vi "UHR-Fleezers Control (host) - 10.7.vi"() -> ()   [LabVIEW 2010] (continued)
            n1703 = case shown="False" w7659 {
              tunnel: w7658 -> [w7665 w7679]
              tunnel: "Chemyx Syringe Pump Serial Port" -> [w7662 w7678]
              frame False {
                n1704 = flat-sequence {
                  tunnel: w7662 -> [w7666]
                  tunnel: [w7666] -> w7663
                  tunnel: w7665 -> [_]
                  tunnel: [w7669] -> w7664
                  tunnel: w7663 -> [w7669]
                  tunnel: w7664 -> [w7670]
                  tunnel: [w7670] -> w7660
                  tunnel: [w7672] -> w7661
                  tunnel: w7660 -> [w7672]
                  tunnel: w7661 -> [w7674]
                  frame #0 {
                    n1705 = call "Write to pump.vi"("string"="enter pump3", "VISA resource name"=w7666) -> ()  [unwired: 1 out]
                  }
                  frame #1 {
                    n1706 = local read "Pump pause delay (ms)"() -> (w7668:u32)
                    n1707 = Wait (ms)(milliseconds to wait=w7668) -> ()  [unwired: 1 out]
                  }
                  frame #2 {
                    n1708 = call "Write to pump.vi"("string"="stop", "VISA resource name"=w7670) -> ()  [unwired: 1 out]
                  }
                  frame #3 {
                    n1709 = Wait (ms)(milliseconds to wait=u32 0) -> ()  [unwired: 1 out]
                  }
                  frame #4 {
                    n1710 = call "Write to pump.vi"("string"="stop", "VISA resource name"=w7674) -> ()  [unwired: 1 out]
                  }
                }
              }
              frame True {
                n1711 = flat-sequence {
                  tunnel: w7678 -> [w7688]
                  tunnel: w7679 -> [w7683]
                  tunnel: w7679 -> [w7690]
                  tunnel: w7678 -> [w7691]
                  tunnel: [w7691] -> w7676
                  tunnel: [w7694] -> w7677
                  tunnel: w7676 -> [w7694]
                  tunnel: w7677 -> [w7695]
                  frame #0 {
                    n1712 = local read "All Pump Parameters"() -> (w7682:T5)
                    n1713 = Unbundle By Name(w7682) -> ("Pump 3"=w7689:T51)
                    n1714 = call "Set pump parameters.vi"("Pump write delay (ms)"=w7683, "Volume (uL)"="Ch 3 Inject Volume (uL)", "Rate (uL/h)"="Ch 3 Inject Rate (ul/h)", "Units"=4.0, "Pump #"=3.0, "Pump Parameters In"=w7689, "VISA resource name"=w7688) -> ("Pump Parameters Out"=w7681:T51)  [unwired: 3 in]
                    n1715 = Bundle By Name(cluster=w7682, "Pump 3"=w7681) -> (w7680:T5)
                    n1716 = local write "All Pump Parameters"(w7680) -> ()
                  }
                  frame #1 {
                    n1717 = Wait (ms)(milliseconds to wait=w7690) -> ()  [unwired: 1 out]
                  }
                  frame #2 {
                    n1718 = call "Write to pump.vi"("string"="start", "VISA resource name"=w7691) -> ()  [unwired: 1 out]
                  }
                  frame #3 {
                    n1719 = Wait (ms)(milliseconds to wait=u32 500) -> ()  [unwired: 1 out]
                  }
                  frame #4 {
                    n1720 = call "Write to pump.vi"("string"="start", "VISA resource name"=w7695) -> ()  [unwired: 1 out]
                  }
                }
              }
            }
          }
          frame Enabled {
            n1721 = call "hamilton_controller.vi"("Open?"=w7697, "valve"=enum16{"A", "B", "C", "D", "ALL"}."A", "action"=T23."MOVE VALVE") -> ()  [unwired: 8 in, 1 out]
          }
        }
      }
      event "Inject Valve B": Value Change {
        n1722 = event-data() -> ()  [unwired: 7 out]
        n1723 = disable-structure shown="Enabled" {
          disable-tunnel: "Inject Valve B" -> [w7701 w7721]
          frame Disabled {
            n1724 = local read "Pump write delay (ms)"() -> (w7703:dbl)
            n1725 = flat-sequence {
              tunnel: w7702 -> [w7716]
              tunnel: w7703 -> [w7712]
              tunnel: w7701 -> [_]
              tunnel: w7703 -> [w7718]
              tunnel: w7702 -> [w7719]
              frame #0 {
                n1726 = local read "All Pump Parameters"() -> (w7711:T5)
                n1727 = Multiply(x=60.0, y="Flush Center Ch Rate (ul/m)") -> (x*y=w7708:dbl)
                n1728 = Unbundle By Name(w7711) -> ("Pump 2"=w7717:T51)
                n1729 = call "Set pump parameters.vi"("Pump write delay (ms)"=w7712, "Volume (uL)"="Flush Center Ch Volume (uL)", "Rate (uL/h)"=w7708, "Units"=3.0, "Pump #"=2.0, "Pump Parameters In"=w7717, "VISA resource name"=w7716) -> ("Pump Parameters Out"=w7710:T51)  [unwired: 3 in]
                n1730 = Bundle By Name(cluster=w7711, "Pump 2"=w7710) -> (w7709:T5)
                n1731 = local write "All Pump Parameters"(w7709) -> ()
                n1732 = Add(x="Flush Center Ch Volume (uL)", y="Total Volume\nFlushed (uL)") -> (x+y=w7705:dbl)
                n1733 = local write "Total Volume\nFlushed (uL)"(w7705) -> ()
              }
              frame #1 {
                n1734 = Wait (ms)(milliseconds to wait=w7718) -> ()  [unwired: 1 out]
              }
              frame #2 {
                n1735 = call "Write to pump.vi"("string"="start", "VISA resource name"=w7719) -> ()  [unwired: 1 out]
              }
            }
            n1736 = local read "Chemyx Syringe Pump Serial Port"() -> (w7702:refnum<visa-resource-name>)
          }
          frame Enabled {
            n1737 = call "hamilton_controller.vi"("Open?"=w7721, "valve"=enum16{"A", "B", "C", "D", "ALL"}."B", "action"=T23."MOVE VALVE") -> ()  [unwired: 8 in, 1 out]
          }
        }
      }
      event "Sample Channel Flow": Value Change {
        n1738 = event-data() -> ()  [unwired: 7 out]
        n1739 = call "hamilton_controller.vi"("Open?"="Sample Channel Flow", "valve"=enum16{"A", "B", "C", "D", "ALL"}."C", "action"=T23."MOVE VALVE") -> ()  [unwired: 8 in, 1 out]
      }
      event "Flip Green Filter": Value Change {
        n1740 = event-data() -> ()  [unwired: 7 out]
        n1741 = Not(x="Flip Green Filter") -> (.not. x?=w7727:bool)
        n1742 = local write "Flip Green Filter"(w7727) -> ()
        n1743 = flat-sequence {
          tunnel: w7735 -> [w7740]
          tunnel: w7734 -> [w7739]
          tunnel: [w7737] -> w7732
          tunnel: [w7736] -> w7731
          tunnel: [w7780] -> w7730
          tunnel: w7732 -> [w7780]
          tunnel: [w7779] -> w7729
          tunnel: w7731 -> [w7779]
          tunnel: w7730 -> [w7784]
          tunnel: w7729 -> [w7783]
          tunnel: [w7782] -> w7733
          frame #0 {
            n1744 = xnode "Read/Write Control"("FPGA VI Reference In"=w7740, "error in"=w7739, "Green Filter Flipper"=TRUE) -> ("FPGA VI Reference Out"=w7737:T19, "error out"=w7736:errorcluster)
          }
          frame #1 {
            n1745 = Wait (ms)(milliseconds to wait=u32 100) -> ()  [unwired: 1 out]
          }
          frame #2 {
            n1746 = xnode "Read/Write Control"("FPGA VI Reference In"=w7784, "error in"=w7783, "Green Filter Flipper"=FALSE) -> ("error out"=w7782:errorcluster)  [unwired: 1 out]
          }
        }
      }
      event "Pump 1 contents", "Pump 3 contents": Value Change {
        n1747 = event-data() -> ()  [unwired: 7 out]
        n1748 = local read "Pump 1 contents"() -> (→"Pump 1 cont disp":string)
        n1749 = local read "Pump 3 contents"() -> (→"Pump 3 cont disp":string)
      }
      event "Reset Trap Pos. FB": Value Change {
        n1750 = event-data() -> ()  [unwired: 7 out]
        n1751 = xnode "Read/Write Control"("FPGA VI Reference In"=w7828, "error in"=w7827, "Trap Pos. FB Reset"="Reset Trap Pos. FB") -> ()  [unwired: 2 out]
      }
      event "Trap Pos. FB ON": Value Change {
        n1752 = event-data() -> ()  [unwired: 7 out]
        n1753 = xnode "Read/Write Control"("FPGA VI Reference In"=w7869, "error in"=w7868, "Force feedback"="Trap Pos. FB ON") -> ()  [unwired: 2 out]
      }
      event "Trap Pos. FB Range", "Trap Pos. FB Gains", "Trap Pos. FB Mult Factor", "Trap Pos. FB Offset Factor", "Trap Pos FB Negate Action", "Trap Pos FB Monitor\nT1 or T2": Value Change {
        n1754 = event-data() -> ()  [unwired: 7 out]
        n1755 = xnode "Read/Write Control"("FPGA VI Reference In"=w7916, "error in"=w7915, "Trap Pos. FB Range"="Trap Pos. FB Range", "Trap Pos. FB Gains"="Trap Pos. FB Gains", "Trap Pos. FB Mult Factor"="Trap Pos. FB Mult Factor", "Trap Pos. FB Offset Factor"="Trap Pos. FB Offset Factor", "Trap Pos FB Negate Action"="Trap Pos FB Negate Action", "Trap Pos FB Monitor T1 or T2"="Trap Pos FB Monitor\nT1 or T2", "AI1 X Scale"="Trap Pos. AI1 X Pre-scale") -> ()  [unwired: 2 out]
      }
      event "Trap Pos FB SP": Value Change {
        n1756 = event-data() -> ()  [unwired: 7 out]
        n1757 = xnode "Read/Write Control"("FPGA VI Reference In"=w8104, "error in"=w8103, "Trap Pos. FB SP"="Trap Pos FB SP") -> ()  [unwired: 2 out]
      }
      event "Set SP to Reading": Value Change {
        n1758 = event-data() -> ()  [unwired: 7 out]
        n1759 = local read "Trap Pos FB Monitor\nT1 or T2"() -> (w8157:bool)
        n1760 = local read "Trap X AI1 (DMA)"() -> (w8160:T13)
        n1761 = local read "Trap X (AI1)"() -> (w8163:T10)
        n1762 = Unbundle By Name(w8163) -> ("Trap 1"=w8162:fxp<+/-,16,1>, "Trap 2"=w8161:fxp<+/-,16,1>)
        n1763 = Unbundle By Name(w8160) -> ("Set 1"=w8159:fxp<+/-,16,1>, "Set 2"=w8158:fxp<+/-,16,1>)
        n1764 = Select(t=w8162, s=w8157, f=w8161) -> (s? t:f=w8156:fxp<+/-,16,1>)
        n1765 = Select(t=w8159, s=w8157, f=w8158) -> (s? t:f=w8155:fxp<+/-,16,1>)
        n1766 = Not(x="Set SP Using...") -> (.not. x?=w8150:bool)
        n1767 = Select(t=w8156, s=w8150, f=w8155) -> (s? t:f=w8151:fxp<+/-,16,1>)
        n1768 = xnode "Read/Write Control"("FPGA VI Reference In"=w8153, "error in"=w8152, "Trap Pos. FB SP"=w8151) -> ()  [unwired: 2 out]
        n1769 = local write "Trap Pos FB SP"(w8151) -> ()
      }
      event "Trap Pos. FB Out Scale 2^n": Value Change {
        n1770 = event-data() -> ()  [unwired: 7 out]
        n1771 = Scale By Power Of 2(n="Trap Pos. FB Out Scale 2^n", x=ext 1.0) -> (x*2^n=w8210:ext)
        n1772 = property on="Trap Pos. FB Mult Factor" class="DigNum (strict)"("Val(Sgnl)"=w8210) -> ()  [unwired: 2 in, 2 out]
      }
      event "Trap Pos FB Int Count": Value Change {
        n1773 = event-data() -> ()  [unwired: 7 out]
        n1774 = xnode "Read/Write Control"("FPGA VI Reference In"=w8215, "error in"=w8214, "Trap Pos FB Int Count"="Trap Pos FB Int Count") -> ()  [unwired: 2 out]
      }
    }
    "error out 2" <- w4481
    n1775 = node-c288() -> ()  [unwired: 1 in, 1 out]
  }
  n1776 = timed-loop "Run Scripts, including: stage motion" {
    timing: w68 -> [_]
    timing-out: [_] -> w67
    tunnel: w16 -> [_]
    stop <- w8254 stop-if-true
    n1777 = node-c288() -> ()  [unwired: 1 in, 1 out]
    n1778 = event shown="[11] \"Got ADig bead\": Value Change" {
      selector: _ -> [_ _ _ _ _ _ _ _ _ _ _ _ _ _ _ _ _]
      dyn-events: _ -> [_ _ _ _ _ _ _ _ _ _ _ _ _ _ _ _ _]
      timeout: 50 -> [_ _ _ _ _ _ _ _ _ _ _ _ _ _ _ _ _]
      tunnel: ["Set Position" "Move to Position" "Move Cap. 1 (DNA Top)" _ "Move Cap. 2 (ADig Bot)" _ "Cal/Data Acq. Spot" "Dump Beads" "Dip for Protein" _ _ "Got ADig bead" "Got DNA bead" "Take Stepping Data" _ "Take Detection Laser\nImage" _] -> _
      tunnel: [_ _ _ _ _ _ _ _ _ _ _ _ _ _ _ _ w8636] -> w8254
      event "Set Position", "Set Position 2", "Set Position 3", "Set Position 4", "Set Position 5", "Set Position 1": Value Change {
        n1779 = event-data() -> ()  [unwired: 1 in, 5 out]
        n1780 = Build Array("Set Position 1", "Set Position 2", "Set Position 3", "Set Position 4", "Set Position 5") -> (w8273:bool[])
        n1781 = Boolean Array To Number(Boolean array=w8273) -> (number=w8272:u32)
        n1782 = Logarithm Base 2(1:w8272) -> (0:w8264:dbl)
        n1783 = call "CONEX_FUNCTIONAL_GLOBAL.vi"("Command"=T22."GET POS") -> ("Current Position"=w8257:dbl[])  [unwired: 8 in, 2 out]
        n1784 = Decrement(x="Position") -> (x-1=w8262:dbl)
        n1785 = Greater Or Equal?(x=w8264, y=0.0) -> (x >= y?=w8265:bool)
        n1786 = Select(t=w8264, s=w8265, f=w8262) -> (s? t:f=w8261:dbl)
        n1787 = Increment(x=w8261) -> (x+1=w8260:dbl)
        n1788 = Build Array (concatenate)(w8260, w8257) -> (w8259:dbl[])
        n1789 = Replace Array Subset(array="Saved Stage Positions", new element=w8259, index (row)=w8261) -> (w8274:dbl[][])  [unwired: 1 in]
        n1790 = local write "Saved Stage Positions"(w8274) -> ()
      }
      event "Move to Position": Value Change {
        n1791 = event-data() -> ()  [unwired: 1 in, 5 out]
        n1792 = flat-sequence {
          frame #0 {
            n1793 = local read "Position"() -> (w8289:dbl)
            n1794 = local read "Saved Stage Positions"() -> (w8287:dbl[][])
            n1795 = Decrement(x=w8289) -> (x-1=w8286:dbl)
            n1796 = Array Subset(array=w8287, index (row)=w8286, length (row)=1 ("length"), index (col)=1 ("index"), length (col)=3 ("length")) -> (w8283:dbl[][])
            n1797 = Reshape Array(w8283, 3 ("dimension size")) -> (w8279:dbl[])
            n1798 = local write "Stage Moving"(TRUE ("Stage Moving")) -> ()
            n1799 = call "CONEX_FUNCTIONAL_GLOBAL.vi"("Axis"=enum16{"X", "Y", "Z", "XY", "XZ", "YZ", "XYZ"}."XYZ", "Position"=w8279, "Command"=T22."ABS MOVE") -> ()  [unwired: 6 in, 3 out]
          }
          frame #1 {
            n1800 = call <vilib>:"Beep.vi"() -> ()  [unwired: 3 in, 9 out]
            n1801 = local write "Stage Moving"(FALSE ("Stage Moving")) -> ()
          }
        }
      }
      event "Move Cap. 1 (DNA Top)": Value Change {
        n1802 = event-data() -> ()  [unwired: 1 in, 5 out]
        n1803 = local write "Move Cap. 1 (DNA Top)"(FALSE ("Move Cap. 1 (DNA Right)")) -> ()
        n1804 = flat-sequence {
          tunnel: ["Cap 1 Samp Flow ON"] -> w8292
          tunnel: w8292 -> [w8311]
          tunnel: [w8311] -> w8291
          tunnel: w8291 -> [w8312]
          frame #0 {
            n1805 = local read "Saved Stage Positions"() -> (w8305:dbl[][])
            n1806 = Array Subset(array=w8305, index (row)=0 ("index"), length (row)=1 ("length"), index (col)=1 ("index"), length (col)=3 ("length")) -> (w8302:dbl[][])
            n1807 = Reshape Array(w8302, 3 ("dimension size")) -> (w8296:dbl[])
            n1808 = case "start flow in central channel to wash" shown="True" "Cap 1 Samp Flow ON" {
              frame False {
              }
              frame True {
                n1809 = call "hamilton_controller.vi"("Open?"=TRUE, "valve"=enum16{"A", "B", "C", "D", "ALL"}."C", "action"=T23."MOVE VALVE") -> ()  [unwired: 8 in, 1 out]
              }
            }
            n1810 = call "CONEX_FUNCTIONAL_GLOBAL.vi"("Axis"=enum16{"X", "Y", "Z", "XY", "XZ", "YZ", "XYZ"}."XYZ", "Position"=w8296, "Command"=T22."ABS MOVE") -> ()  [unwired: 6 in, 3 out]
            n1811 = local write "Stage Moving"(TRUE ("Stage Moving")) -> ()
          }
          frame #1 {
            # "should replace this frame\nwith code that \ncontinuously polls the\nCONEX controllers to\ndetermine when the \nmotors have finished \nmoving. once the move \nis finished, proceed to\nnext frame"
            n1812 = Wait (ms)(milliseconds to wait=u32 5000) -> ()  [unwired: 1 out]
          }
          frame #2 {
            n1813 = local write "Stage Moving"(FALSE ("Stage Moving")) -> ()
            n1814 = case "stop flow" shown="False" w8312 {
              frame False {
              }
              frame True {
                n1815 = call "hamilton_controller.vi"("Open?"=FALSE, "valve"=enum16{"A", "B", "C", "D", "ALL"}."C", "action"=T23."MOVE VALVE") -> ()  [unwired: 8 in, 1 out]
              }
            }
            n1816 = case shown="True" TRUE {
              tunnel: "Cap 1 T ON" -> [w8321 w8322]
              frame False {
                n1817 = property on="Trap 1 (ON/OFF)" class="Bool (strict)"("Val(Sgnl)"=w8321) -> ()  [unwired: 2 in, 2 out]
              }
              frame True {
                n1818 = property on="Trap 2 (ON/OFF)" class="Bool (strict)"("Val(Sgnl)"=w8322) -> ()  [unwired: 2 in, 2 out]
              }
            }
            n1819 = call <vilib>:"Beep.vi"() -> ()  [unwired: 3 in, 9 out]
            n1820 = case shown="True" "Cap 1 Flow ON" {
              frame False {
              }
              frame True {
                n1821 = property on="Inject Top" class="Bool (strict)"("Val(Sgnl)"=TRUE ("Value (Signaling)")) -> ()  [unwired: 2 in, 2 out]
              }
            }
          }
        }
      }
      event Timeout {
        n1822 = event-data() -> ()  [unwired: 1 in, 2 out]
      }
      event "Move Cap. 2 (ADig Bot)": Value Change {
        n1823 = event-data() -> ()  [unwired: 1 in, 5 out]
        n1824 = local write "Move Cap. 2 (ADig Bot)"(FALSE ("Move Cap. 2 (ADig Left)")) -> ()
        n1825 = flat-sequence {
          tunnel: ["Cap 2 Samp Flow ON"] -> w8324
          tunnel: w8324 -> [w8343]
          tunnel: [w8343] -> w8323
          tunnel: w8323 -> [w8344]
          frame #0 {
            n1826 = local read "Saved Stage Positions"() -> (w8337:dbl[][])
            n1827 = case shown="True" "Cap 2 Samp Flow ON" {
              frame False {
              }
              frame True {
                n1828 = call "hamilton_controller.vi"("Open?"=TRUE, "valve"=enum16{"A", "B", "C", "D", "ALL"}."C", "action"=T23."MOVE VALVE") -> ()  [unwired: 8 in, 1 out]
              }
            }
            n1829 = Array Subset(array=w8337, index (row)=1 ("index"), length (row)=1 ("length"), index (col)=1 ("index"), length (col)=3 ("length")) -> (w8334:dbl[][])
            n1830 = Reshape Array(w8334, 3 ("dimension size")) -> (w8328:dbl[])
            n1831 = local write "Stage Moving"(TRUE ("Stage Moving")) -> ()
            n1832 = call "CONEX_FUNCTIONAL_GLOBAL.vi"("Axis"=enum16{"X", "Y", "Z", "XY", "XZ", "YZ", "XYZ"}."XYZ", "Position"=w8328, "Command"=T22."ABS MOVE") -> ()  [unwired: 6 in, 3 out]
          }
          frame #1 {
            n1833 = Wait (ms)(milliseconds to wait=u32 5000) -> ()  [unwired: 1 out]
          }
          frame #2 {
            n1834 = local write "Stage Moving"(FALSE ("Stage Moving")) -> ()
            n1835 = case shown="True" TRUE {
              tunnel: "Cap 2 T ON" -> [w8353 w8354]
              frame False {
                n1836 = property on="Trap 2 (ON/OFF)" class="Bool (strict)"("Val(Sgnl)"=w8353) -> ()  [unwired: 2 in, 2 out]
              }
              frame True {
                n1837 = property on="Trap 1 (ON/OFF)" class="Bool (strict)"("Val(Sgnl)"=w8354) -> ()  [unwired: 2 in, 2 out]
              }
            }
            n1838 = call <vilib>:"Beep.vi"() -> ()  [unwired: 3 in, 9 out]
            n1839 = case shown="True" w8344 {
              frame False {
              }
              frame True {
                n1840 = call "hamilton_controller.vi"("Open?"=FALSE, "valve"=enum16{"A", "B", "C", "D", "ALL"}."C", "action"=T23."MOVE VALVE") -> ()  [unwired: 8 in, 1 out]
              }
            }
            n1841 = case shown="True" "Cap 2 Flow ON" {
              frame False {
              }
              frame True {
                n1842 = property on="Inject Bottom" class="Bool (strict)"("Val(Sgnl)"=TRUE ("Value (Signaling)")) -> ()  [unwired: 2 in, 2 out]
              }
            }
          }
        }
      }
      event "+z", "-z": Value Change {
        n1843 = event-data() -> ()  [unwired: 1 in, 5 out]
        n1844 = flat-sequence {
          frame #0 {
            w8356 = 0.0 ("element")
            n1845 = Divide(x="z nudge increment (um)", y=1000.0) -> (x/y=w8369:dbl)
            n1846 = Boolean To (0,1)(Boolean="+z") -> (0, 1=w8362:i16)
            n1847 = Boolean To (0,1)(Boolean="-z") -> (0, 1=w8363:i16)
            n1848 = Multiply(x=w8362, y=w8369) -> (x*y=w8366:dbl)
            n1849 = Multiply(x=w8363, y=w8369) -> (x*y=w8364:dbl)
            n1850 = Negate(x=w8364) -> (-x=w8365:dbl)
            n1851 = Add(x=w8366, y=w8365) -> (x+y=w8357:dbl)
            n1852 = Build Array(w8356, w8356, w8357) -> (w8355:dbl[])
            n1853 = call "CONEX_FUNCTIONAL_GLOBAL.vi"("Axis"=enum16{"X", "Y", "Z", "XY", "XZ", "YZ", "XYZ"}."Z", "Position"=w8355, "Command"=T22."REL MOVE") -> ()  [unwired: 6 in, 3 out]
            n1854 = local write "Stage Moving"(TRUE ("Stage Moving")) -> ()
          }
          frame #1 {
            n1855 = local write "Stage Moving"(FALSE ("Stage Moving")) -> ()
            n1856 = call <vilib>:"Beep.vi"() -> ()  [unwired: 3 in, 9 out]
          }
        }
      }
      event "Cal/Data Acq. Spot": Value Change {
        # "wait for calibration file\nto be written"
        # "signal save cal true\nthis tells the data \nacquisition loop to\nstart sending the data\nto a calibration file"
        # "separate traps to\nthe desired trap delta"
        # "move stage to data acquisition spot"
        # "CHANGE FISH FOR TETHER BACK\nTO TRUE VALUE HERE."
        n1857 = event-data() -> ()  [unwired: 1 in, 5 out]
        n1858 = flat-sequence {
          tunnel: ["Cal @ (MHz)"] -> w8372
          tunnel: w8372 -> [w8394]
          tunnel: w8372 -> [w8415]
          frame #0 {
            n1859 = local read "Saved Stage Positions"() -> (w8380:dbl[][])
            n1860 = Array Subset(array=w8380, index (row)=2 ("index"), length (row)=1 ("length"), index (col)=1 ("index"), length (col)=3 ("length")) -> (w8383:dbl[][])
            n1861 = Reshape Array(w8383, 3 ("dimension size")) -> (w8376:dbl[])
            n1862 = local write "Stage Moving"(TRUE ("Stage Moving")) -> ()
            n1863 = call "CONEX_FUNCTIONAL_GLOBAL.vi"("Axis"=enum16{"X", "Y", "Z", "XY", "XZ", "YZ", "XYZ"}."XYZ", "Position"=w8376, "Command"=T22."ABS MOVE") -> ()  [unwired: 6 in, 3 out]
          }
          frame #1 {
            n1864 = property on="Trap Delta (MHz)" class="DigNum (strict)"("Val(Sgnl)"="Cal @ (MHz)") -> ()  [unwired: 2 in, 2 out]
            n1865 = local write "Stage Moving"(FALSE ("Stage Moving")) -> ()
            n1866 = call <vilib>:"Beep.vi"() -> ()  [unwired: 3 in, 9 out]
          }
          frame #2 {
            n1867 = Wait (ms)(milliseconds to wait=u32 100) -> ()  [unwired: 1 out]
          }
          frame #3 {
            n1868 = property on="Save Calibration" class="Bool (strict)"("Val(Sgnl)"=TRUE ("Value (Signaling)")) -> ()  [unwired: 2 in, 2 out]
          }
          frame #4 {
            n1869 = Wait (ms)(milliseconds to wait=u32 4000) -> ()  [unwired: 1 out]
          }
          frame #5 {
            n1870 = while {
              stop <- w8391 stop-if-true
              n1871 = local read "Saving..."() -> (w8392:bool)
              n1872 = Wait (ms)(milliseconds to wait=u32 100) -> ()  [unwired: 1 out]
              n1873 = Not(x=w8392) -> (.not. x?=w8391:bool)
            }
          }
          frame #6 {
            n1874 = case shown="True" "W/ Offset 1" {
              tunnel: w8394 -> [_ w8396]
              frame False {
              }
              frame True {
                n1875 = stacked-sequence {
                  tunnel: w8396 -> [_ _ _ _ _ _ _ w8413]
                  frame #0 {
                    n1876 = property on="Trap Delta (MHz)" class="DigNum (strict)"("Val(Sgnl)"="Offset 1 Start (MHz)") -> ()  [unwired: 2 in, 2 out]
                    n1877 = Replace Array Subset(array=u32[] [0] ("Index Values"), new element="Offset 1 Set", index=0) -> (w8397:u32[])
                    n1878 = property on="Saved AOD Raster Scan Parameter Sets" class="Arr (strict)"("Index Values"=w8397) -> ()  [unwired: 2 in, 2 out]
                  }
                  frame #1 {
                    n1879 = Wait (ms)(milliseconds to wait=u32 200) -> ()  [unwired: 1 out]
                  }
                  frame #2 {
                    n1880 = property on="Load parameters" class="Bool (strict)"("Val(Sgnl)"=TRUE ("Value (Signaling)")) -> ()  [unwired: 2 in, 2 out]
                  }
                  frame #3 {
                    n1881 = Wait (ms)(milliseconds to wait=u32 200) -> ()  [unwired: 1 out]
                  }
                  frame #4 {
                    n1882 = property on="Trap Raster Scan" class="Bool (strict)"("Val(Sgnl)"=TRUE ("Value (Signaling)")) -> ()  [unwired: 2 in, 2 out]
                  }
                  frame #5 {
                    n1883 = Wait (ms)(milliseconds to wait=u32 2000) -> ()  [unwired: 1 out]
                  }
                  frame #6 {
                    n1884 = while {
                      stop <- w8410 stop-if-true
                      n1885 = local read "Raster Scanning..."() -> (w8412:bool)
                      n1886 = local read "Saving..."() -> (w8408:bool)
                      n1887 = Wait (ms)(milliseconds to wait=u32 100) -> ()  [unwired: 1 out]
                      n1888 = Not(x=w8408) -> (.not. x?=w8407:bool)
                      n1889 = Not(x=w8412) -> (.not. x?=w8409:bool)
                      n1890 = And(x=w8409, y=w8407) -> (x .and. y?=w8410:bool)
                    }
                  }
                  frame #7 {
                    n1891 = property on="Trap Delta (MHz)" class="DigNum (strict)"("Val(Sgnl)"=w8413) -> ()  [unwired: 2 in, 2 out]
                  }
                }
              }
            }
          }
          frame #7 {
            n1892 = local read "Save ave N"() -> (w8414:dbl)
            n1893 = case shown="True" "W/ Offset 2" {
              tunnel: w8415 -> [_ w8421]
              tunnel: w8414 -> [_ w8420]
              frame False {
                n1894 = Multiply(x="Cal read wait (s)", y=u32 1000 ("milliseconds to wait")) -> (x*y=w8418:u32)
                n1895 = Wait (ms)(milliseconds to wait=w8418) -> ()  [unwired: 1 out]
              }
              frame True {
                n1896 = stacked-sequence {
                  tunnel: w8421 -> [_ _ _ _ _ _ _ _ _ w8442 _ _]
                  tunnel: w8420 -> [_ _ _ _ _ _ _ _ _ w8440 _ _]
                  frame #0 {
                    n1897 = property on="Save ave N" class="DigNum (strict)"("Val(Sgnl)"=1.0 ("Value (Signaling)")) -> ()  [unwired: 2 in, 2 out]
                  }
                  frame #1 {
                    n1898 = Wait (ms)(milliseconds to wait=u32 500) -> ()  [unwired: 1 out]
                  }
                  frame #2 {
                    n1899 = property on="Trap Delta (MHz)" class="DigNum (strict)"("Val(Sgnl)"="Offset 2 Start (MHz)") -> ()  [unwired: 2 in, 2 out]
                    n1900 = Replace Array Subset(array=u32[] [0] ("Index Values"), new element="Offset 2 Set", index=0) -> (w8426:u32[])
                    n1901 = property on="Saved AOD Raster Scan Parameter Sets" class="Arr (strict)"("Index Values"=w8426) -> ()  [unwired: 2 in, 2 out]
                  }
                  frame #3 {
                    n1902 = Wait (ms)(milliseconds to wait=u32 500) -> ()  [unwired: 1 out]
                  }
                  frame #4 {
                    n1903 = property on="Load parameters" class="Bool (strict)"("Val(Sgnl)"=TRUE ("Value (Signaling)")) -> ()  [unwired: 2 in, 2 out]
                  }
                  frame #5 {
                    n1904 = Wait (ms)(milliseconds to wait=u32 500) -> ()  [unwired: 1 out]
                  }
                  frame #6 {
                    n1905 = property on="Trap Raster Scan" class="Bool (strict)"("Val(Sgnl)"=TRUE ("Value (Signaling)")) -> ()  [unwired: 2 in, 2 out]
                  }
                  frame #7 {
                    n1906 = Wait (ms)(milliseconds to wait=u32 2000) -> ()  [unwired: 1 out]
                  }
                  frame #8 {
                    n1907 = while {
                      stop <- w8435 stop-if-true
                      n1908 = local read "Raster Scanning..."() -> (w8438:bool)
                      n1909 = local read "Saving..."() -> (w8436:bool)
                      n1910 = Wait (ms)(milliseconds to wait=u32 100) -> ()  [unwired: 1 out]
                      n1911 = Not(x=w8436) -> (.not. x?=w8434:bool)
                      n1912 = Not(x=w8438) -> (.not. x?=w8437:bool)
                      n1913 = And(x=w8437, y=w8434) -> (x .and. y?=w8435:bool)
                    }
                  }
                  frame #9 {
                    n1914 = property on="Trap Delta (MHz)" class="DigNum (strict)"("Val(Sgnl)"=w8442) -> ()  [unwired: 2 in, 2 out]
                    n1915 = property on="Saved AOD Raster Scan Parameter Sets" class="Arr (strict)"("Index Values"=u32[] [0]) -> ()  [unwired: 2 in, 2 out]
                    n1916 = property on="Save ave N" class="DigNum (strict)"("Val(Sgnl)"=w8440) -> ()  [unwired: 2 in, 2 out]
                  }
                  frame #10 {
                    n1917 = Wait (ms)(milliseconds to wait=u32 500) -> ()  [unwired: 1 out]
                  }
                  frame #11 {
                    n1918 = property on="Load parameters" class="Bool (strict)"("Val(Sgnl)"=TRUE ("Value (Signaling)")) -> ()  [unwired: 2 in, 2 out]
                  }
                }
              }
            }
          }
          frame #8 {
            n1919 = property on="Read Cal" class="Bool (strict)"("Val(Sgnl)"=TRUE ("Value (Signaling)")) -> ()  [unwired: 2 in, 2 out]
          }
          frame #9 {
            n1920 = Wait (ms)(milliseconds to wait=u32 500) -> ()  [unwired: 1 out]
          }
          frame #10 {
            n1921 = property on="Fish for Tether" class="Bool (strict)"("Val(Sgnl)"=FALSE ("Value (Signaling)")) -> ()  [unwired: 2 in, 2 out]
          }
        }
        n1922 = local write "Cal/Data Acq. Spot"(FALSE ("Cal/Data Acq. Spot")) -> ()
      }
      event "Dump Beads": Value Change {
        # "SCRIPT TO REMOVE BOTH BEADS FROM THE TRAPS. TURNS ON LIGHT WHICH INDICATES THAT STAGE IS MOVING. THEN STOPS SAVING DATA. \nSETS Sample Channel Flow TO TRUE. STOPS INTERLACING GREEN FLUORESCENCE. TURNS OFF Tether INDICATOR BECAUSE WE ARE THROWING IT\nAWAY. SHUTS OFF TRAP POSITION FEEDBACK."
        n1923 = event-data() -> ()  [unwired: 1 in, 5 out]
        n1924 = flat-sequence {
          frame #0 {
            w8449 = FALSE ("Fl. Triggered...")
            w8450 = TRUE ("Stage Moving")
            n1925 = local read "Saving..."() -> (w8451:bool)
            n1926 = local write "Fl. Triggered..."(w8449) -> ()
            n1927 = local write "Stage Moving"(w8450) -> ()
            n1928 = local write "Tether"(w8449) -> ()
            n1929 = property on="Green Laser ON/Interlacing" class="Bool (strict)"("Val(Sgnl)"=w8449) -> ()  [unwired: 2 in, 2 out]
            n1930 = property on="Trap Pos. FB ON" class="Bool (strict)"("Val(Sgnl)"=w8449) -> ()  [unwired: 2 in, 2 out]
            n1931 = property on="Sample Channel Flow" class="Bool (strict)"("Val(Sgnl)"=w8450) -> ()  [unwired: 2 in, 2 out]
            n1932 = local write "Stop Saving"(w8451) -> ()
          }
          frame #1 {
            # "MOVES TO THE DUMP BEADS POSITION"
            n1933 = local read "Saved Stage Positions"() -> (w8455:dbl[][])
            n1934 = Array Subset(array=w8455, index (row)=3 ("index"), length (row)=1 ("length"), index (col)=1 ("index"), length (col)=3 ("length")) -> (w8458:dbl[][])
            n1935 = Reshape Array(w8458, 3 ("dimension size")) -> (w8453:dbl[])
            n1936 = call "CONEX_FUNCTIONAL_GLOBAL.vi"("Axis"=enum16{"X", "Y", "Z", "XY", "XZ", "YZ", "XYZ"}."XYZ", "Position"=w8453, "Command"=T22."ABS MOVE") -> ()  [unwired: 6 in, 3 out]
          }
          frame #2 {
            n1937 = Wait (ms)(milliseconds to wait=u32 5000) -> ()  [unwired: 1 out]
          }
          frame #3 {
            w8463 = FALSE ("Value (Signaling)")
            # "TURNS TRAPS OFF SO THAT\nBEADS REMAIN AT DUMP \nBEADS POSITION"
            n1938 = property on="Trap 1 (ON/OFF)" class="Bool (strict)"("Val(Sgnl)"=w8463) -> ()  [unwired: 2 in, 2 out]
            n1939 = property on="Trap 2 (ON/OFF)" class="Bool (strict)"("Val(Sgnl)"=w8463) -> ()  [unwired: 2 in, 2 out]
            n1940 = call <vilib>:"Beep.vi"() -> ()  [unwired: 3 in, 9 out]
          }
          frame #4 {
            # "MOVES STAGE BACK TO THE\nANTIDIG CAPILARY BY CALLING\nTHE Move Cap. 2 SCRIPT"
            n1941 = property on="Move Cap. 2 (ADig Bot)" class="Bool (strict)"("Val(Sgnl)"=TRUE ("Value (Signaling)")) -> ()  [unwired: 2 in, 2 out]
          }
        }
      }
      event "Dip for Protein": Value Change {
        n1942 = event-data() -> ()  [unwired: 1 in, 5 out]
        n1943 = flat-sequence {
          frame #0 {
            n1944 = case shown="True" "Move Trap Before?" {
              frame False {
              }
              frame True {
                n1945 = property on="Trap Delta (MHz)" class="DigNum (strict)"("Val(Sgnl)"="Dip Trap Delta 1 (MHz)") -> ()  [unwired: 2 in, 2 out]
              }
            }
          }
          frame #1 {
            n1946 = local read "Saved Stage Positions"() -> (w8471:dbl[][])
            n1947 = Array Subset(array=w8471, index (row)=4 ("index"), length (row)=1 ("length"), index (col)=1 ("index"), length (col)=3 ("length")) -> (w8474:dbl[][])
            n1948 = Reshape Array(w8474, 3 ("dimension size")) -> (w8469:dbl[])
            n1949 = call "CONEX_FUNCTIONAL_GLOBAL.vi"("Axis"=enum16{"X", "Y", "Z", "XY", "XZ", "YZ", "XYZ"}."XYZ", "Position"=w8469, "Command"=T22."ABS MOVE") -> ()  [unwired: 6 in, 3 out]
          }
          frame #2 {
            n1950 = Multiply(x="Duration (s)", y=1000.0) -> (x*y=w8478:dbl)
            n1951 = Wait (ms)(milliseconds to wait=w8478) -> ()  [unwired: 1 out]
          }
          frame #3 {
            n1952 = local read "Saved Stage Positions"() -> (w8484:dbl[][])
            n1953 = Array Subset(array=w8484, index (row)=2 ("index"), length (row)=1 ("length"), index (col)=1 ("index"), length (col)=3 ("length")) -> (w8487:dbl[][])
            n1954 = Reshape Array(w8487, 3 ("dimension size")) -> (w8482:dbl[])
            n1955 = call "CONEX_FUNCTIONAL_GLOBAL.vi"("Axis"=enum16{"X", "Y", "Z", "XY", "XZ", "YZ", "XYZ"}."XYZ", "Position"=w8482, "Command"=T22."ABS MOVE") -> ()  [unwired: 6 in, 3 out]
          }
          frame #4 {
            n1956 = case shown="True" "Move Trap After?" {
              frame False {
              }
              frame True {
                n1957 = property on="Trap Delta (MHz)" class="DigNum (strict)"("Val(Sgnl)"="Dip Trap Delta 2 (MHz)") -> ()  [unwired: 2 in, 2 out]
              }
            }
          }
          frame #5 {
            n1958 = case shown="True" "Green ON After?" {
              frame False {
              }
              frame True {
                n1959 = property on="Green Laser ON/Interlacing" class="Bool (strict)"("Val(Sgnl)"=TRUE ("Value (Signaling)")) -> ()  [unwired: 2 in, 2 out]
              }
            }
          }
          frame #6 {
            n1960 = Wait (ms)(milliseconds to wait=u32 500) -> ()  [unwired: 1 out]
          }
          frame #7 {
            n1961 = case shown="True" "Save Data After?" {
              frame False {
              }
              frame True {
                n1962 = property on="Start Saving" class="Bool (strict)"("Val(Sgnl)"=TRUE ("Value (Signaling)")) -> ()  [unwired: 2 in, 2 out]
              }
            }
          }
        }
      }
      event "Profile": Value Change {
        n1963 = event-data() -> ()  [unwired: 1 in, 5 out]
        n1964 = flat-sequence {
          tunnel: [w8500] -> w8499
          tunnel: w8499 -> [w8504]
          tunnel: [w8503] -> w8498
          tunnel: w8498 -> [w8510]
          frame #0 {
            w8501 = 0.0 ("element")
            n1965 = Build Array(w8501, "Y change (mm)", w8501) -> (w8500:dbl[])
          }
          frame #1 {
            # "move to new position and start saving"
            n1966 = local write "Stage Moving"(TRUE ("Stage Moving")) -> ()
            n1967 = local write "Start Saving"(TRUE ("Start Saving")) -> ()
            n1968 = call "CONEX_FUNCTIONAL_GLOBAL.vi"("Axis"=enum16{"X", "Y", "Z", "XY", "XZ", "YZ", "XYZ"}."Y", "Position"=w8504, "Command"=T22."REL MOVE") -> ()  [unwired: 6 in, 3 out]
            n1969 = Negate(x=w8504) -> (-x=w8503:dbl[])
          }
          frame #2 {
            # "go back to start"
            n1970 = call "CONEX_FUNCTIONAL_GLOBAL.vi"("Axis"=enum16{"X", "Y", "Z", "XY", "XZ", "YZ", "XYZ"}."Y", "Position"=w8510, "Command"=T22."REL MOVE") -> ()  [unwired: 6 in, 3 out]
          }
          frame #3 {
            # "stop saving"
            n1971 = local write "Stop Saving"(TRUE ("Stop Saving")) -> ()
            n1972 = local write "Stage Moving"(FALSE ("Stage Moving")) -> ()
          }
        }
      }
      event "Move to Position 1", "Move to Position 2", "Move to Position 3", "Move to Position 4", "Move to Position 5", "Lower Ch. Cap.": Value Change {
        n1973 = event-data() -> ()  [unwired: 1 in, 5 out]
        n1974 = Or(x="Move to Position 5", y="Lower Ch. Cap.") -> (x .or. y?=w8515:bool)
        n1975 = Build Array("Move to Position 1", "Move to Position 2", "Move to Position 3", "Move to Position 4", w8515) -> (w8518:bool[])
        n1976 = Boolean Array To Number(Boolean array=w8518) -> (number=w8517:u32)
        n1977 = Logarithm Base 2(1:w8517) -> (0:w8516:dbl)
        n1978 = flat-sequence {
          tunnel: w8516 -> [w8528]
          frame #0 {
            n1979 = local read "Saved Stage Positions"() -> (w8533:dbl[][])
            n1980 = Array Subset(array=w8533, index (row)=w8528, length (row)=1 ("length"), index (col)=1 ("index"), length (col)=3 ("length")) -> (w8530:dbl[][])
            n1981 = Reshape Array(w8530, 3 ("dimension size")) -> (w8525:dbl[])
            n1982 = local write "Stage Moving"(TRUE ("Stage Moving")) -> ()
            n1983 = call "CONEX_FUNCTIONAL_GLOBAL.vi"("Axis"=enum16{"X", "Y", "Z", "XY", "XZ", "YZ", "XYZ"}."XYZ", "Position"=w8525, "Command"=T22."ABS MOVE") -> ()  [unwired: 6 in, 3 out]
          }
          frame #1 {
            n1984 = local write "Stage Moving"(FALSE ("Stage Moving")) -> ()
            n1985 = call <vilib>:"Beep.vi"() -> ()  [unwired: 3 in, 9 out]
          }
        }
      }
      event "Got ADig bead": Value Change {
        n1986 = event-data() -> ()  [unwired: 1 in, 5 out]
        n1987 = property on="Move Cap. 1 (DNA Top)" class="Bool (strict)"("Val(Sgnl)"=TRUE ("Value (Signaling)")) -> ()  [unwired: 2 in, 2 out]
        n1988 = property on="Inject Top" class="Bool (strict)"("Val(Sgnl)"=FALSE ("Value (Signaling)")) -> ()  [unwired: 2 in, 2 out]
      }
      event "Got DNA bead": Value Change {
        n1989 = event-data() -> ()  [unwired: 1 in, 5 out]
        n1990 = property on="Cal/Data Acq. Spot" class="Bool (strict)"("Val(Sgnl)"=TRUE ("Value (Signaling)")) -> ()  [unwired: 2 in, 2 out]
        n1991 = property on="Inject Bottom" class="Bool (strict)"("Val(Sgnl)"=FALSE ("Value (Signaling)")) -> ()  [unwired: 2 in, 2 out]
      }
      event "Take Stepping Data": Value Change {
        n1992 = event-data() -> ()  [unwired: 1 in, 5 out]
        n1993 = local read "Save ave N"() -> (w8550:dbl)
        n1994 = flat-sequence {
          tunnel: w8550 -> [w8552]
          tunnel: [w8552] -> w8545
          tunnel: [w8554] -> w8546
          tunnel: w8545 -> [w8554]
          tunnel: [w8556] -> w8547
          tunnel: w8546 -> [w8556]
          tunnel: [w8559] -> w8548
          tunnel: w8547 -> [w8559]
          tunnel: [w8561] -> w8549
          tunnel: w8548 -> [w8561]
          tunnel: [w8563] -> w8543
          tunnel: w8549 -> [w8563]
          tunnel: w8543 -> [w8566]
          tunnel: [w8566] -> w8542
          tunnel: w8542 -> [w8567]
          tunnel: [w8567] -> w8544
          tunnel: w8544 -> [w8573]
          frame #0 {
            n1995 = property on="Save ave N" class="DigNum (strict)"("Val(Sgnl)"="Save ave factor") -> ()  [unwired: 2 in, 2 out]
          }
          frame #1 {
            n1996 = Wait (ms)(milliseconds to wait=u32 100) -> ()  [unwired: 1 out]
          }
          frame #2 {
            n1997 = local read "Offset 2 Start (MHz)"() -> (w8558:dbl)
            n1998 = property on="Saved AOD Raster Scan Parameter Sets" class="Arr (strict)"("Index Values"=u32[] [2]) -> ()  [unwired: 2 in, 2 out]
            n1999 = property on="Trap Delta (MHz)" class="DigNum (strict)"("Val(Sgnl)"=w8558) -> ()  [unwired: 2 in, 2 out]
          }
          frame #3 {
            n2000 = property on="Load parameters" class="Bool (strict)"("Val(Sgnl)"=TRUE ("Value (Signaling)")) -> ()  [unwired: 2 in, 2 out]
          }
          frame #4 {
            n2001 = Wait (ms)(milliseconds to wait=u32 100) -> ()  [unwired: 1 out]
          }
          frame #5 {
            n2002 = property on="Trap Raster Scan" class="Bool (strict)"("Val(Sgnl)"=TRUE ("Value (Signaling)")) -> ()  [unwired: 2 in, 2 out]
          }
          frame #6 {
            n2003 = Wait (ms)(milliseconds to wait=u32 1000) -> ()  [unwired: 1 out]
          }
          frame #7 {
            n2004 = while {
              stop <- w8570 stop-if-true
              n2005 = local read "Raster Scanning..."() -> (w8572:bool)
              n2006 = local read "Saving..."() -> (w8571:bool)
              n2007 = Not(x=w8571) -> (.not. x?=w8568:bool)
              n2008 = Not(x=w8572) -> (.not. x?=w8569:bool)
              n2009 = And(x=w8569, y=w8568) -> (x .and. y?=w8570:bool)
            }
          }
          frame #8 {
            n2010 = property on="Save ave N" class="DigNum (strict)"("Val(Sgnl)"=w8573) -> ()  [unwired: 2 in, 2 out]
          }
        }
      }
      event "Step Size (nm)": Value Change {
        n2011 = event-data() -> ()  [unwired: 1 in, 5 out]
        n2012 = flat-sequence {
          frame #0 {
            n2013 = property on="Saved AOD Raster Scan Parameter Sets" class="Arr (strict)"("Index Values"=u32[] [1]) -> ()  [unwired: 2 in, 2 out]
          }
          frame #1 {
            n2014 = Multiply(x="N Steps", y="Step Size (nm)") -> (x*y=w8575:dbl)
            n2015 = property on="Scan Speed AOD (nm/s) 2" class="DigNum (strict)"("Value"="Step Size (nm)") -> ()  [unwired: 2 in, 2 out]
            n2016 = property on="Step Size AOD (nm) 2" class="DigNum (strict)"("Value"="Step Size (nm)") -> ()  [unwired: 2 in, 2 out]
            n2017 = property on="Scan Range AOD (nm) 2" class="DigNum (strict)"("Value"=w8575) -> ()  [unwired: 2 in, 2 out]
          }
        }
      }
      event "Take Detection Laser\nImage": Value Change {
        n2018 = event-data() -> ()  [unwired: 1 in, 5 out]
        n2019 = flat-sequence {
          tunnel: [w8603] -> w8593
          tunnel: [w8602] -> w8586
          tunnel: [w8601] -> w8578
          tunnel: [w8606] -> w8594
          tunnel: w8593 -> [w8606]
          tunnel: [w8605] -> w8587
          tunnel: w8586 -> [w8605]
          tunnel: [w8604] -> w8579
          tunnel: w8578 -> [w8604]
          tunnel: [w8610] -> w8595
          tunnel: w8594 -> [w8610]
          tunnel: [w8609] -> w8588
          tunnel: w8587 -> [w8609]
          tunnel: [w8608] -> w8580
          tunnel: w8579 -> [w8608]
          tunnel: [w8616] -> w8596
          tunnel: w8595 -> [w8616]
          tunnel: [w8615] -> w8589
          tunnel: w8588 -> [w8615]
          tunnel: [w8614] -> w8581
          tunnel: w8580 -> [w8614]
          tunnel: [w8620] -> w8597
          tunnel: w8596 -> [w8620]
          tunnel: [w8619] -> w8590
          tunnel: w8589 -> [w8619]
          tunnel: [w8618] -> w8582
          tunnel: w8581 -> [w8618]
          tunnel: [w8624] -> w8598
          tunnel: w8597 -> [w8624]
          tunnel: [w8623] -> w8591
          tunnel: w8590 -> [w8623]
          tunnel: [w8622] -> w8583
          tunnel: w8582 -> [w8622]
          tunnel: [w8628] -> w8599
          tunnel: w8598 -> [w8628]
          tunnel: [w8627] -> w8592
          tunnel: w8591 -> [w8627]
          tunnel: [w8626] -> w8584
          tunnel: w8583 -> [w8626]
          tunnel: w8599 -> [w8634]
          tunnel: w8592 -> [w8633]
          tunnel: [w8631] -> w8585
          tunnel: w8584 -> [w8631]
          tunnel: w8585 -> [w8635]
          frame #0 {
            n2020 = local read "Green Laser ON/Interlacing"() -> (w8603:bool)
            n2021 = local read "Green laser mode"() -> (w8602:enum32{"Laser ON", "Laser OFF", "Interlace"})
            n2022 = local read "Green FB On/Off"() -> (w8601:bool)
          }
          frame #1 {
            n2023 = property on="Green FB On/Off" class="Bool (strict)"("Val(Sgnl)"=FALSE ("Value (Signaling)")) -> ()  [unwired: 2 in, 2 out]
          }
          frame #2 {
            n2024 = property on="Green Laser ON/Interlacing" class="Bool (strict)"("Val(Sgnl)"=TRUE ("Value (Signaling)")) -> ()  [unwired: 2 in, 2 out]
            n2025 = property on="Flip Green Filter" class="Bool (strict)"("Val(Sgnl)"=TRUE ("Value (Signaling)")) -> ()  [unwired: 2 in, 2 out]
            n2026 = property on="Green laser mode" class="RadioBtnsControl (strict)"("Val(Sgnl)"=enum32{"Laser ON", "Laser OFF", "Interlace"}."Laser ON" ("Value (Signaling)")) -> ()  [unwired: 2 in, 2 out]
          }
          frame #3 {
            n2027 = Wait (ms)(milliseconds to wait=u32 500) -> ()  [unwired: 1 out]
          }
          frame #4 {
            n2028 = property on="Confocal Image" class="Bool (strict)"("Val(Sgnl)"=TRUE ("Value (Signaling)")) -> ()  [unwired: 2 in, 2 out]
          }
          frame #5 {
            n2029 = Wait (ms)(milliseconds to wait=u32 2000) -> ()  [unwired: 1 out]
          }
          frame #6 {
            n2030 = while {
              stop <- w8629 stop-if-true
              n2031 = local read "Saving..."() -> (w8630:bool)
              n2032 = Not(x=w8630) -> (.not. x?=w8629:bool)
            }
          }
          frame #7 {
            n2033 = property on="Flip Green Filter" class="Bool (strict)"("Val(Sgnl)"=TRUE ("Value (Signaling)")) -> ()  [unwired: 2 in, 2 out]
            n2034 = property on="Green Laser ON/Interlacing" class="Bool (strict)"("Val(Sgnl)"=w8634) -> ()  [unwired: 2 in, 2 out]
            n2035 = property on="Green laser mode" class="RadioBtnsControl (strict)"("Val(Sgnl)"=w8633) -> ()  [unwired: 2 in, 2 out]
          }
          frame #8 {
            n2036 = property on="Green FB On/Off" class="Bool (strict)"("Val(Sgnl)"=w8635) -> ()  [unwired: 2 in, 2 out]
          }
        }
      }
      event "Stop All": Value Change {
        n2037 = event-data() -> ()  [unwired: 1 in, 5 out]
        n2038 = local read "Stop All"() -> (w8636:bool)
      }
    }
    n2039 = node-c288() -> ()  [unwired: 1 in, 1 out]
  }
  n2040 = timed-loop "Mouse control: trap position (AOM deflection), set confocal spot from image" {
    tunnel: [w8638] -> w31
    tunnel: w16 -> [w8637]
    timing: w75 -> [_]
    timing-out: [_] -> w74
    stop <- w8638 stop-if-true
    n2041 = node-c288() -> ()  [unwired: 2 out]
    n2042 = event shown="[0] \"Pane\": Mouse Down" {
      selector: _ -> [_ _]
      dyn-events: _ -> [_ _]
      timeout: _ -> [_ _]
      tunnel: w8637 -> [w8641 _]
      event Mouse Down {
        n2043 = event-data() -> ("Time"=w8643:u32, "Coords"=w8642:T7, "Button"=w8644:u16)  [unwired: 6 out]
        n2044 = case shown="1" w8644 {
          tunnel: w8643 -> [_ _ w8747]
          tunnel: w8642 -> [_ w8681 w8745]
          tunnel: w8641 -> [_ _ w8743]
          frame 0, Default {
          }
          frame 1 {
            n2045 = property on="APD 2" class="ImageControl"() -> ("Displayed Image Position"=w8651:cluster{"Left":i32, "Top":i32})  [unwired: 2 in, 2 out]
            n2046 = property on="APD 1" class="ImageControl"() -> ("Displayed Image Position"=w8680:cluster{"Left":i32, "Top":i32})  [unwired: 2 in, 2 out]
            n2047 = property on="Detection Laser X" class="ImageControl"() -> ("Displayed Image Position"=w8677:cluster{"Left":i32, "Top":i32})  [unwired: 2 in, 2 out]
            n2048 = property on="Detection Laser Y" class="ImageControl"() -> ("Displayed Image Position"=w8676:cluster{"Left":i32, "Top":i32})  [unwired: 2 in, 2 out]
            n2049 = property on="APD 2" class="ImageControl"() -> ("Displayed Image Size"=w8650:cluster{"Width":u32, "Height":u32})  [unwired: 2 in, 2 out]
            n2050 = property on="APD 1" class="ImageControl"() -> ("Displayed Image Size"=w8678:cluster{"Width":u32, "Height":u32})  [unwired: 2 in, 2 out]
            n2051 = property on="Detection Laser X" class="ImageControl"() -> ("Displayed Image Size"=w8679:cluster{"Width":u32, "Height":u32})  [unwired: 2 in, 2 out]
            n2052 = property on="Detection Laser Y" class="ImageControl"() -> ("Displayed Image Size"=w8675:cluster{"Width":u32, "Height":u32})  [unwired: 2 in, 2 out]
            n2053 = Unbundle By Name(w8650) -> ("Width"=w8647:u32, "Height"=w8646:u32)
            n2054 = Unbundle By Name(w8651) -> ("Left"=w8649:i32, "Top"=w8648:i32)
            n2055 = Unbundle By Name(w8678) -> ("Width"=w8672:u32, "Height"=w8671:u32)
            n2056 = Unbundle By Name(w8679) -> ("Width"=w8668:u32, "Height"=w8667:u32)
            n2057 = Unbundle By Name(w8675) -> ("Width"=w8664:u32, "Height"=w8663:u32)
            n2058 = Unbundle By Name(w8680) -> ("Left"=w8674:i32, "Top"=w8673:i32)
            n2059 = Unbundle By Name(w8677) -> ("Left"=w8670:i32, "Top"=w8669:i32)
            n2060 = Unbundle By Name(w8676) -> ("Left"=w8666:i32, "Top"=w8665:i32)
            n2061 = Bundle("Left"=w8649, "Top"=w8648, "Width"=w8647, "Height"=w8646) -> (w8645:T52)  [unwired: 1 in]
            n2062 = Bundle("Left"=w8674, "Top"=w8673, "Width"=w8672, "Height"=w8671) -> (w8662:T52)  [unwired: 1 in]
            n2063 = Bundle("Left"=w8670, "Top"=w8669, "Width"=w8668, "Height"=w8667) -> (w8661:T52)  [unwired: 1 in]
            n2064 = Bundle("Left"=w8666, "Top"=w8665, "Width"=w8664, "Height"=w8663) -> (w8660:T52)  [unwired: 1 in]
            n2065 = Build Cluster Array(w8645, w8662, w8661, w8660) -> (w8659:T53)
            n2066 = for {
              tunnel: w8681 -> [w8692]
              tunnel: w8659 -> [w8693] mode=indexing
              shift-right: [w8690] -> w8657
              shift-left: TRUE -> [w8691]
              shift-right: [w8689] -> w8655
              shift-left: _ -> [w8685]
              shift-right: [w8688] -> w8654
              shift-left: _ -> [w8684]
              shift-right: [w8687] -> w8653
              shift-left: _ -> [w8683]
              shift-right: [w8686] -> w8652
              shift-left: _ -> [w8682]
              n2067 = case shown="True" w8691 {
                selector: w8691 -> [w8698 _]
                tunnel: w8693 -> [_ w8707]
                tunnel: w8692 -> [_ w8705]
                tunnel: [w8698 w8703] -> w8690
                tunnel: [w8697 w8702] -> w8689
                tunnel: [w8696 w8701] -> w8688
                tunnel: [w8695 w8700] -> w8687
                tunnel: [w8694 w8699] -> w8686
                tunnel: w8685 -> [w8697 _]
                tunnel: w8684 -> [w8696 _]
                tunnel: w8683 -> [w8695 _]
                tunnel: w8682 -> [w8694 _]
                frame False {
                }
                frame True {
                  n2068 = Unbundle(w8707) -> (w8706:T52)
                  n2069 = call "isclickinwindow.vi"("Image Param"=w8706, "Point32"=w8705) -> ("4 Y"=w8699:i32, "3 Height"=w8700:i32, "2 X"=w8701:i32, "1 Width"=w8702:i32, "In image?"=w8704:bool)  [unwired: 1 in]
                  n2070 = Not(x=w8704) -> (.not. x?=w8703:bool)
                }
              }
            }
            n2071 = Not(x=w8657) -> (.not. x?=w8656:bool)
            n2072 = case shown="True" w8656 {
              tunnel: w8654 -> [_ w8720]
              tunnel: w8652 -> [_ w8719]
              tunnel: w8655 -> [_ w8718]
              tunnel: w8653 -> [_ w8717]
              frame False {
              }
              frame True {
                w8713 = FALSE ("Get Point")
                n2073 = local read "Scan lines (y)"() -> (w8722:u64)
                n2074 = local read "Actual MCL Inc (V)"() -> (w8714:dbl)
                n2075 = local read "Scan steps (MCL)"() -> (w8721:u64)
                n2076 = Divide "Y Pix/step"(x=w8717, y=w8722) -> (x/y=w8729:dbl)
                n2077 = Divide "Y V/pix"(x=w8714, y=w8729) -> (x/y=w8728:dbl)
                n2078 = Divide "Y half step offset"(x=w8714, y=2.0) -> (x/y=w8730:dbl)
                n2079 = Divide "X pix/step"(x=w8718, y=w8721) -> (x/y=w8727:dbl)
                n2080 = Negate(x=w8730) -> (-x=w8731:dbl)
                n2081 = local read "Initial Y"() -> (w8737:dbl)
                n2082 = Multiply(x=w8719, y=w8728) -> (x*y=w8738:dbl)